vi "RetriggerableHost_20230407a.vi"() -> ()   [LabVIEW 2021]
doc: "Use this VI as a template to design an application that acquires data using advanced triggering logic from the NI PXIe-5170R/5171R."
uses:
  <instrlib>/_niInstr/Multirecord Acquisition/Interface/v1/Host/Public/Requested Record Info.ctl
  Controls/Queue_Data_Type.ctl
  <instrlib>/HSAI-RIO/Types/v1/Host/Typedefs/Temp Source.ctl
  <vilib>/FPGAPlugInAG/PXIe-5172 (8CH - 325T)/niLvFpga_Open_PXIe-5172 (8CH - 325T).vi
  <vilib>/rvi/interface/common/dynamic/niFpgaDynamicAddResources.vi
  <vilib>/FPGAPlugInAG/Dynamic/niLvFpga_Close_Dynamic.vi
  <vilib>/rvi/interface/nirviOpenFPGA/nirviOpenFPGA.xnode
  FPGA Bitfiles/Multirecord Acquisition_20220927.lvbitx
  <vilib>/rvi/interface/nirviCloseFPGA/nirviCloseFPGA.xnode
  Device Session/Device Session.lvclass
  <instrlib>/HSAI-RIO/Types/v1/Host/niHSAI Types v1 Host.lvlib
  <vilib>/Utility/TDMS File Viewer/NI_TDMS File Viewer.lvlib
  <instrlib>/_niInstr/Multirecord Acquisition/Interface/v1/Host/niInstr Multirecord Acquisition v1 Host.lvclass
panel:
  out "LoopCount":i32
  out "requested records info":T1[](array[typedef])
  out "error out 2":errorcluster
  out "appended path":path
  out "Trigger":bool
  in  "trigger level lo (V)":dbl=-0.25
  in  "trigger level hi (V)":dbl=0.25
  out "actual sample rate":dbl=200000000.0 format="%#_6p"
  in  "onboard sample clock rate":dbl(ring)=200000000.0 items=["250 MHz"=250000000.0, "200 MHz"=200000000.0, "150 MHz"=150000000.0]
  in  "impedance":enum8{"Default", "1 mega ohm", "50 ohm"}(ring)=enum."50 ohm"
  in  "vertical offset (V)":dbl format="%.2p"
  out "Graph":T2(graph)
  out "fpga temperature (°C)":dbl(slide)=84.16040039062506 scale=0.0..96.0 scale format="%#_6p"
  out "power consumption (W)":dbl(slide)=28.75 scale=0.0..38.25 scale format="%#_6p"
  in  "decimation factor":u16=1
  in  "coupling":enum8{"Default", "DC", "AC"}(ring)
  in  "bandwidth":T3(ring)
  in  "pretrigger samples":u64=500
  in  "number of samples":u64=1000
  in  "RIO Device":tag="PXI1Slot2"
  in  "channel(s)":string="0,1"
  in  "vertical range (Vpp)":dbl=1.0 format="%.2p"
  out "error out":errorcluster
  in  "stop":bool
  # "RIO Device"
  # "Vertical Settings"
  # "Trigger Settings"
  # "System Monitor"
  # "Acquisition Settings"
  # "Clocking"
  # "DSP"
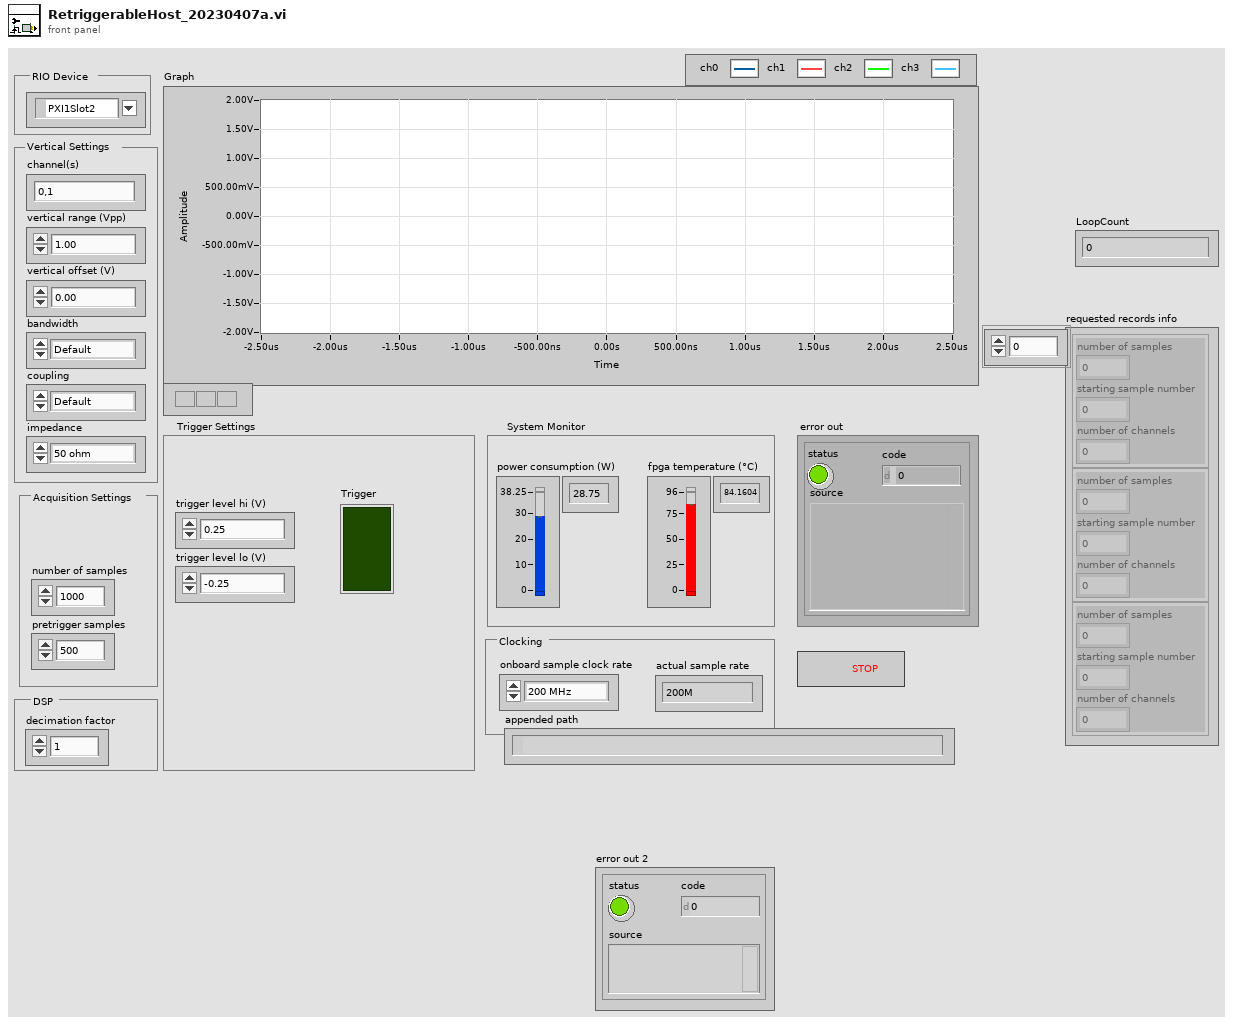
[diagram p1: front panel]
types:
  T1 = typedef "niInstr Multirecord Acquisition v1 Host.lvclass/Requested Record Info.ctl" = cluster{"number of samples":u64, "starting sample number":u64, "number of channels":u64, "timestamps":u64[]}
  T2 = cluster{"relativeX":dbl, "sample rate":dbl, "data in":dbl[]}[]
  T3 = enum8{"Default", "Full Bandwidth", "Anti-alias Filter", "80 MHz FIR Filter", "40 MHz FIR Filter", "20 MHz FIR Filter"}
  T4 = enum16{"Immediate", "A", "B", "OR", "AND", "A THEN B", "B THEN A", "High Resolution"}
  T5 = typedef "niHSAI Types v1 Host.lvlib/Temp Source.ctl" = enum8{"Device Temperature", "Thermal Shutdown Margin", "FPGA Temperature", "FPGA Temperature Limit"}
  T6 = typedef "Queue_Data_Type.ctl" = cluster{"date/time string":string, "data":dbl[][]}
  T7 = enum16{"open", "open or create", "create or replace", "create", "open (read-only)"}
  T8 = cluster{"date/time string":string, "data":dbl[][]}
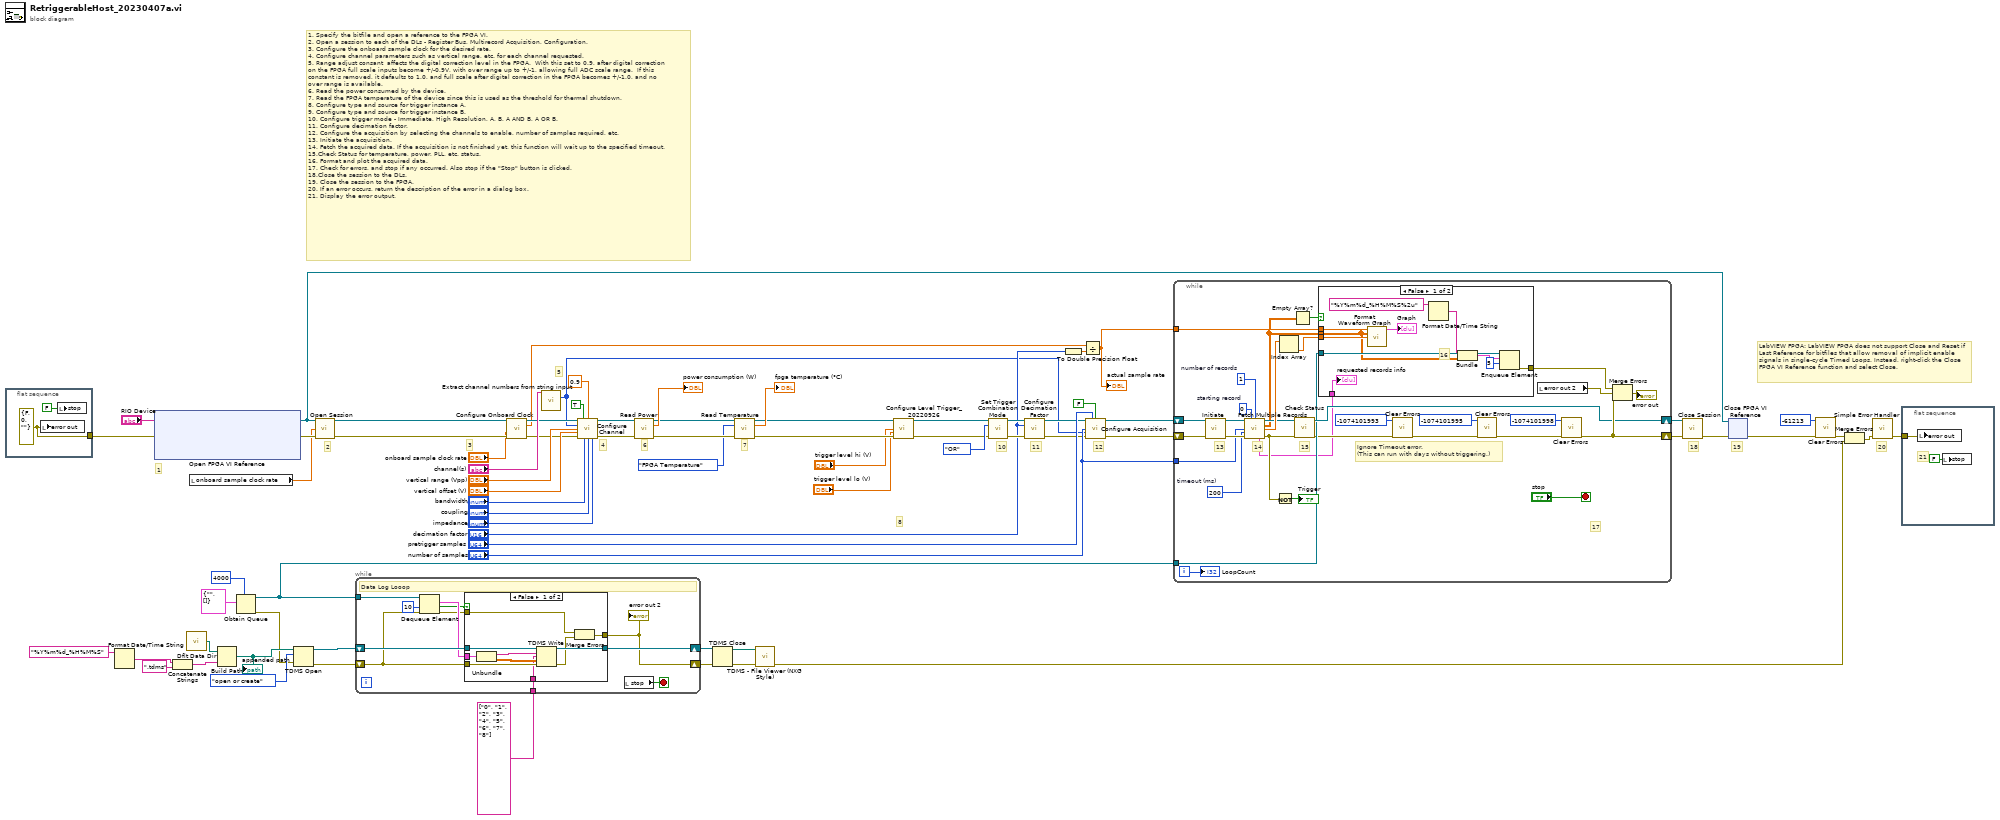
[diagram p0: block diagram]
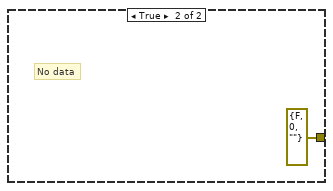
[diagram p2: hidden frame]
diagram:
  # "4"
  # "5"
  # "7"
  # "6"
  # "11"
  # "3"
  # "10"
  # "8"
  # "12"
  # "LabVIEW FPGA: LabVIEW FPGA does not support Close and Reset if Last Reference for bitfiles that allow removal of implicit enable signals in single-cycle Timed Loops. Instead, right-click the Close FPGA VI Reference function and select Close."
  # "20"
  # "19"
  # "18"
  # "1. Specify the bitfile and open a reference to the FPGA VI.\n2. Open a session to each of the DLs - Register Bus, Multirecord Acquisition, Configuration.\n3. Configure the onboard sample clock for the desired rate.\n4. Configure channel parameters such as vertical range, etc. for each channel requested.\n5. Range adjust consant  affects the digital correction level in the FPGA.  With this set to 0.9, after digital correction\non the FPGA full scale inputs become +/-0.9V, with over range up to +/-1, allowing full ADC scale range.  If this \nconstant is removed, it defaults to 1.0, and full scale after digital correction in the FPGA becomes +/-1.0, and no\nover range is available.  \n6. Read the power consumed by the device.\n7. Read the FPGA temperature of the device since this is used as the threshold for thermal shutdown.\n8. Configure type and source for trigger instance A.\n9. Configure type and source for trigger instance B.\n10. Configure trigger mode - Immediate, High Resolution, A, B, A AND B, A OR B.\n11. Configure decimation factor.\n12. Configure the acquisition by selecting the channels to enable, number of samples required, etc.\n13. Initiate the acquisition.\n14. Fetch the acquired data. If the acquisition is not finished yet, this function will wait up to the specified timeout.\n15.Check Status for temperature, power, PLL, etc. status. \n16. Format and plot the acquired data.\n17. Check for errors, and stop if any occurred. Also stop if the \"Stop\" button is clicked.\n18.Close the session to the DLs.\n19. Close the session to the FPGA.\n20. If an error occurs, return the description of the error in a dialog box.\n21. Display the error output."
  # "2"
  # "1"
  n1 = flat-sequence {
    tunnel: [w75] -> w63
    frame #0 {
      w75 = errorcluster {"status"=FALSE, "code"=0, "source"=""} ("error out")
      n2 = local write "error out"(w75) -> ()
      n3 = local write "stop"(FALSE ("stop")) -> ()
    }
  }
  n4 = Format Date/Time String(time format string (%c)="%Y%m%d_%H%M%S") -> (date/time string=w61:string)  [unwired: 2 in]
  n5 = xnode "Open FPGA VI Reference"("error in"=w63, "resource name"="RIO Device") -> ("FPGA VI Reference Out"=w66:refnum<k20>, "error out"=w68:errorcluster)
  n6 = Concatenate Strings(w61, ".tdms" ("string")) -> (w60:string)
  n7 = call <vilib>:"Dflt Data Dir.vi"() -> ("App:Default Data Directory"=w62:path)
  n8 = local read "onboard sample clock rate"() -> (w65:dbl)
  n9 = Build Path(base path=w62, name or relative path=w60) -> (appended path=w57:path)
  "appended path" <- w57
  n10 = Obtain Queue(max queue size (-1, unlimited)=4000, element data type=T6 {"date/time string"="", "data"=[]} ("cluster")) -> (queue out=w47:refnum<queue>, error out=w55:errorcluster)  [unwired: 3 in, 1 out]
  n11 = TDMS Open(8:w55, 10:T7."open or create" ("operation (0:open)"), 11:w57) -> (0:w53:errorcluster, 3:w50:refnum<k34>)  [unwired: 4 in]
  n12 = call "Open Session.vi"("fpga reference in"=w66, "adc clock rate (Hz)"=w65, "error in"=w68) -> ("device session out"=w71:refnum<class "Device Session.lvclass">, "error out"=w70:errorcluster)  [unwired: 11 in]
  n13 = while {
    shift-right: [w78] -> w52
    shift-left: w53 -> [w83]
    shift-right: [w85] -> w49
    shift-left: w50 -> [w86]
    tunnel: w47 -> [w84]
    tunnel: string[] ["0", "1", "2", "3", "4", "5", "6", "7", "8"] ("channel name(s) in (Untitled)") -> [w76]
    stop <- w80 stop-if-true
    # "Data Log Looop"
    n14 = Dequeue Element(queue=w84, timeout in ms (-1)=10, error in (no error)=w83) -> (element=w82:T6, timed out?=w77:bool, error out=w81:errorcluster)  [unwired: 1 out]
    n15 = case shown="False" w77 {
      tunnel: w86 -> [w96 w98]
      tunnel: [w95 w98] -> w85
      tunnel: w83 -> [w94 _]
      tunnel: w82 -> [w93 _]
      tunnel: w81 -> [w92 w97]
      tunnel: [w90 w97] -> w78
      tunnel: w76 -> [w87 _]
      frame False {
        n16 = Unbundle(w93) -> ("date/time string"=w89:string, "data"=w88:dbl[][])
        n17 = TDMS Write(0:w96, 5:w89, 7:w87, 9:w88, 11:w94) -> (4:w95:refnum<k34>, 15:w91:errorcluster)  [unwired: 1 in, 2 out]
        n18 = Merge Errors(w92, w91) -> (w90:errorcluster)
      }
      frame True {
        # "Timed out. No data."
      }
    }
    "error out 2" <- w78
    n19 = local read "stop"() -> (w80:bool)
  }
  n20 = call "Configure Onboard Clock.vi"("device session in"=w71, "adc clock rate (Hz)"="onboard sample clock rate", "error in"=w70) -> ("device session out"=w32:refnum<class "Device Session.lvclass">, "actual adc clock rate (Hz)"=w24:dbl, "error out"=w31:errorcluster)  [unwired: 9 in, 1 out]
  n21 = call "Extract channel numbers from string input.vi"("channel input"="channel(s)") -> ("array of chans"=w6:u32[])  [unwired: 13 in, 1 out]
  n22 = call "Configure Channel.vi"("device session in"=w32, "enable channel (T)"=TRUE ("enable channel"), "range adjust"=0.9, "channels"=w6, "vertical range (Vpp)"="vertical range (Vpp)", "vertical offset (V)"="vertical offset (V)", "error in"=w31, "bandwidth"="bandwidth", "coupling"="coupling", "impedance"="impedance") -> ("device session out"=w18:refnum<class "Device Session.lvclass">, "error out"=w17:errorcluster)  [unwired: 4 in]
  n23 = call "Read Power.vi"("device session in"=w18, "error in"=w17) -> ("device session out"=w19:refnum<class "Device Session.lvclass">, "power (W)"=→"power consumption (W)":dbl, "error out"=w20:errorcluster)  [unwired: 11 in]
  n24 = TDMS Close(8:w52, 11:w49) -> (0:w51:errorcluster, 3:w48:path)
  n25 = call "Read Temperature.vi"("device session in"=w19, "source"=Temp_Source."FPGA Temperature", "error in"=w20) -> ("device session out"=w16:refnum<class "Device Session.lvclass">, "temperature (°C)"=→"fpga temperature (°C)":dbl, "error out"=w15:errorcluster)  [unwired: 10 in]
  n26 = call <vilib>:"TDMS - File Viewer (NXG Style).vi"("error in"=w51, "file in"=w48) -> ("error out"=w45:errorcluster)  [unwired: 8 in, 1 out]
  n27 = call "Configure Level Trigger_20220926.vi"("device session in"=w16, "trigger level hi (V)"="trigger level hi (V)", "trigger level lo (V)"="trigger level lo (V)", "error in"=w15) -> ("device session out"=w5:refnum<class "Device Session.lvclass">, "error out"=w4:errorcluster)  [unwired: 10 in]
  n28 = call "Set Trigger Combination Mode.vi"("device session in"=w5, "mode"=T4."OR", "error in"=w4) -> ("device session out"=w29:refnum<class "Device Session.lvclass">, "error out"=w28:errorcluster)  [unwired: 11 in]
  n29 = call "Configure Decimation Factor.vi"("device session in"=w29, "decimation factor"="decimation factor", "error in"=w28) -> ("device session out"=w26:refnum<class "Device Session.lvclass">, "error out"=w27:errorcluster)  [unwired: 11 in]
  n30 = To Double Precision Float(number="decimation factor") -> (double precision float=w30:dbl)
  n31 = Divide(x=w24, y=w30) -> (x/y=w8:dbl)
  "actual sample rate" <- w8
  n32 = call "Configure Acquisition.vi"("device session in"=w26, "pretrigger samples"="pretrigger samples", "number of records is finite (T)"=FALSE, "number of samples"="number of samples", "channels to store"=w6, "error in"=w27) -> ("device session out"=w37:refnum<class "Device Session.lvclass">, "error out"=w38:errorcluster)  [unwired: 7 in, 1 out]
  n33 = while {
    tunnel: w47 -> [w127]
    tunnel: "number of samples" -> [w122]
    tunnel: w8 -> [w118]
    shift-right: [w129] -> w73
    shift-left: w38 -> [w126]
    shift-right: [w128] -> w72
    shift-left: w37 -> [w123]
    i -> [w99]
    stop <- "stop" stop-if-true
    w106 = u64 0  # starting record
    w105 = u64 1  # number of records
    w103 = 200  # timeout (ms)
    # "Ignore Timeout error.\n(This can run with days without triggering.)"
    # "15"
    # "17"
    # "14"
    # "13"
    n34 = call "Initiate.vi"("device session in"=w123, "error in"=w126) -> ("device session out"=w124:refnum<class "Device Session.lvclass">, "error out"=w125:errorcluster)  [unwired: 12 in]
    n35 = call "Fetch Multiple Records.vi"("device session in"=w124, "starting record"=w106, "number of records"=w105, "number of samples"=w122, "timeout (ms)"=w103, "error in"=w125) -> ("device session out"=w119:refnum<class "Device Session.lvclass">, "data"=w110:dbl[][], "relativeX (samples)"=w121:dbl[], "requested records info"=w100:T1[], "error out"=w111:errorcluster)  [unwired: 5 in]
    n36 = Not(x=w111) -> (.not. x?=→"Trigger":bool)
    n37 = Index Array(array=w121) -> (element=w104:dbl)  [unwired: 1 in]
    n38 = Empty Array?(array=w110) -> (empty?=w109:bool)
    n39 = call "Check Status.vi"("device session in"=w119, "error in"=w111) -> ("device session out"=w128:refnum<class "Device Session.lvclass">, "error out"=w120:errorcluster)  [unwired: 12 in]
    n40 = case shown="False" w109 {
      tunnel: w110 -> [w136 _]
      tunnel: w104 -> [w140 _]
      tunnel: w118 -> [w138 _]
      tunnel: w127 -> [w137 _]
      tunnel: [w131 errorcluster {"status"=FALSE, "code"=0, "source"=""} ("error out")] -> w101
      tunnel: w100 -> [w130 _]
      frame False {
        # "16"
        n41 = call "Format Waveform Graph.vi"("sample rate (Hz)"=w138, "data in"=w136, "relativeX (samples)"=w140) -> ("waveform out"=→"Graph":T2)  [unwired: 12 in]
        n42 = Format Date/Time String(time format string (%c)="%Y%m%d_%H%M%S%2u") -> (date/time string=w132:string)  [unwired: 2 in]
        n43 = Bundle("date/time string"=w132, "data"=w136) -> (w133:T8)  [unwired: 1 in]
        n44 = Enqueue Element(queue=w137, element=w133, timeout in ms (-1)=5) -> (error out=w131:errorcluster)  [unwired: 1 in, 2 out]
        "requested records info" <- w130
      }
      frame True {
        # "No data"
      }
    }
    n45 = call <vilib>:"Clear Errors.vi"("error in (no error)"=w120, "specific error code to clear (0: all)"=-1074101993) -> ("error out"=w115:errorcluster)  [unwired: 4 in, 1 out]
    n46 = call <vilib>:"Clear Errors.vi"("error in (no error)"=w115, "specific error code to clear (0: all)"=-1074101995) -> ("error out"=w113:errorcluster)  [unwired: 4 in, 1 out]
    n47 = local read "error out 2"() -> (w107:errorcluster)
    n48 = call <vilib>:"Clear Errors.vi"("error in (no error)"=w113, "specific error code to clear (0: all)"=-1074101998) -> ("error out"=w129:errorcluster)  [unwired: 4 in, 1 out]
    n49 = Merge Errors(w101, w107, w129) -> (→"error out":errorcluster)
    "LoopCount" <- w99
  }
  n50 = call "Close Session.vi"("device session in"=w72, "error in"=w73) -> ("error out"=w67:errorcluster)  [unwired: 13 in]
  n51 = xnode "Close FPGA VI Reference"("FPGA VI Reference In"=w66, "error in"=w67) -> ("error out"=w41:errorcluster)
  n52 = call <vilib>:"Clear Errors.vi"("error in (no error)"=w41, "specific error code to clear (0: all)"=-61213) -> ("error out"=w40:errorcluster)  [unwired: 4 in, 1 out]
  n53 = Merge Errors(w40, w45) -> (w46:errorcluster)
  n54 = call <vilib>:"Simple Error Handler.vi"("error in (no error)"=w46) -> ("error out"=w64:errorcluster)  [unwired: 4 in, 4 out]
  n55 = flat-sequence {
    tunnel: w64 -> [w143]
    frame #0 {
      # "21"
      n56 = local write "error out"(w143) -> ()
      n57 = local write "stop"(FALSE ("stop")) -> ()
    }
  }
